vi "reconstruct 3D oblique image without config-2 (SubVI).vi"(0 "correction":T2={"vibration removal"=FALSE, "x correct fast/slow"=TRUE, "y correct fast/slow"=TRUE, "z correct fast/slow"=TRUE}, 1 "auto z adjust":T1={"margin"=100.0, "auto z adj"=FALSE, "average"=10, "use given ofst"=FALSE, "given ofst"=10}, 5 "image in":u16[][][](array[numeric])=array4x300x2304[2764800 elements], 7 "config in":T3={"xy cut pos correct"=[[0.0, 0.0, 0.0, 0.0], [0.0, 0.0, 0.0, 0.0], [0.0, 0.0, 0.0, 0.0], [0.0, 0.0, 0.0, 0.0], [0.0, 0.0, 0.0, 0.0], [0.0, 0.0, 0.0, 0.0], [0.0, 0.0, 0.0, 0.0], [0.0, 0.0, 0.0, 0.0], [0.0, 0.0, 0.0, 0.0], [0.0, 0.0, 0.0, 0.0], [0.0, 0.0, 0.0, 0.0], [0.0, 0.0, 0.0, 0.0], [0.0, 0.0, 0.0, 0.0], [0.0, 0.0, 0.0, 0.0], [0.0, 0.0, 0.0, 0.0], [0.0, 0.0, 0.0, 0.0], [0.0, 0.0, 0.0, 0.0], [0.0, 0.0, 0.0, 0.0], [0.0, 0.0, 0.0, 0.0], [0.0, 0.0, 0.0, 0.0], [0.0, 0.0, 0.0, 0.0], [0.0, 0.0, 0.0, 0.0], [0.0, 0.0, 0.0, 0.0], [0.0, 0.0, 0.0, 0.0]], "3D reconst config"={"xyz pos"=[46, 31, 52], "color 4"={"color array"=[0, 8388736, 16711680, 16776960, 16776960, 16711680, 16448250, 16448250], "num of colors"=4, "max"=7000.900000000023, "min"=100.0}, "autogain"=TRUE, "zoom"=1.0, "slice(T)/stack(F)"=FALSE, "xy cut mag"=0.9999999999999872, "xy cut ofst"=10.0, "z/xy comp"=0.9999999999999996, "y shift comp"=2.0, "max plot"=TRUE, "oblique angle [deg]"=45.0, "voxel size z [um]"=0.2909342537087903, "voxel size xy[um]"=0.20475, "reverse v"=FALSE, "reverse h"=TRUE, "3D reconstruction"=TRUE, "reverse z"=FALSE}, "xy cut pos"=[[0.0, 1.037506591193278, 0.966249270369417, 0.9158940969875857], [92.08631074928655, 92.74282819847565, 92.97750230838835, 92.67727146331777], [184.28758330950427, 185.01250778668418, 185.4134489785189, 184.69137479417213], [276.0489606758347, 276.53636075026884, 276.69217675847005, 276.4860055768869], [368.07921566607354, 368.89819980674065, 368.8136411193633, 368.38419699919905], [461.798744208641, 461.9849633403935, 462.2490904762467, 462.24814037863575], [554.7781467122519, 555.268397079519, 555.2332434679125, 554.7296917340917], [647.2882009960379, 647.5846314506646, 647.6995932615935, 647.5152743250628], [740.8889673372312, 741.2737568696792, 741.2034496464664, 740.8557139208467], [833.9643296995517, 834.1876026381326, 834.4726319214276, 834.3510194272217], [926.4886354475025, 926.7024074099736, 926.5560923778821, 926.5332900352184], [1019.2086613033152, 1019.556397028935, 1019.5734987859327, 1019.5449958576031], [1112.8274794991178, 1113.0498023400878, 1112.7296194451865, 1112.9329403339368], [1205.8866902020513, 1205.9931011344815, 1205.9531970348203, 1205.9037919590492], [1298.9126474886007, 1298.899346122047, 1299.058012423081, 1299.116918474962], [1392.299641867323, 1392.3689989929248, 1391.9509560440924, 1392.082069514408], [1485.6457820487744, 1485.6942370269344, 1485.3132478849304, 1485.3569523750357], [1578.3297041953701, 1578.9007128595708, 1578.61948396672, 1578.8503576861888], [1671.6273893986595, 1671.6549422293779, 1671.4050665576897, 1671.3604119699735], [1764.8661685500688, 1764.862368159625, 1764.8129630838534, 1765.1844512497485], [1857.8854751533427, 1857.8854751533427, 1857.6869047526473, 1857.7192080714206], [1951.1917112351302, 1951.1964617231852, 1951.2800703129517, 1951.4168843689333], [2043.5326481441634, 2043.787274303907, 2043.6352586861497, 2043.5982048793212], [2136.2422229262547, 2136.4265418627856, 2136.2099196074814, 2136.124410822493]], "AOD scan speed ratio"=5.0, "Nx"=93.5, "stack method"=enum."0pad to x and rot", "y shift"=3}, 9 "cropcalib":bool, 11 "cropcalib data":dbl[][][](array[numeric])=[[[330.8512624722854, 1176.151016996622, 0.0, 0.009428316830650669], [328.5787621076082, 1180.3546677235079, 0.0, 0.009179659527843352], [329.1155115826025, 1185.5118549945614, 0.0, 0.008879926465064643], [328.4474666338575, 1190.066406913501, 0.0, 0.00862012495571322]], [[327.58384877552515, 1179.3399452115818, 0.0, 0.009239326761173557], [330.64586772559215, 1183.570509586454, 0.0, 0.008992065492687374], [329.1182426075196, 1188.7090456628334, 0.0, 0.008697068994156926], [331.0833292234464, 1193.2988555935556, 0.0, 0.008438543533451089]], [[328.7041098476068, 1182.569513173517, 0.0, 0.009050212846350443], [330.5655883182281, 1186.770481635967, 0.0, 0.008807670479919528], [328.3880581820918, 1191.9068661319957, 0.0, 0.00851645191863399], [330.8192081039448, 1196.484526211637, 0.0, 0.008261875826756079]], [[329.0291138405168, 1185.8638941976924, 0.0, 0.00885968095793796], [330.2239592659729, 1190.0021055331606, 0.0, 0.008623760711384792], [329.88360431477196, 1195.207928124911, 0.0, 0.00833239920230058], [329.0055546600167, 1200.7794531816844, 0.0, 0.008027295813293513]], [[330.24527413712724, 1189.0833512123208, 0.0, 0.008675809944263788], [328.9577860583197, 1193.1902259931223, 0.0, 0.0084446078534114], [328.4487732377894, 1198.4548030016394, 0.0, 0.008153748883619465], [330.0763524036554, 1204.0443558848656, 0.0, 0.00785175048715124]], [[327.9606329363599, 1192.2041314919686, 0.0, 0.008499777889598343], [330.446114732459, 1196.4188076408827, 0.0, 0.008265497412007088], [331.55926553798633, 1201.6905041902264, 0.0, 0.007978069360316281], [330.71140004975507, 1207.1845836973916, 0.0, 0.0076851779540676735]], [[329.5691345378466, 1195.4239688330229, 0.0, 0.008320438746162742], [330.7306447795087, 1200.618390032539, 0.0, 0.008036017910836857], [329.65318996509365, 1204.906703846507, 0.0, 0.007805785611196943], [330.4225359020906, 1210.364940978633, 0.0, 0.0075187501899264125]], [[328.35008836956763, 1198.6407415088522, 0.0, 0.008143589762204376], [328.90402303435104, 1203.8024115267247, 0.0, 0.007864676757548733], [328.8872850578613, 1208.09777539, 0.0, 0.007637156351356103], [328.3105695920642, 1213.5593257233536, 0.0, 0.007353896502053807]], [[328.6451967358637, 1127.9703327325547, 0.0, 0.012550072767244045], [328.19424909379455, 1133.085548853325, 0.0, 0.012195479564778025], [328.3679132256721, 1137.3419122345406, 0.0, 0.011904528149263727], [329.8664011804312, 1142.824068114119, 0.0, 0.011535328382056603]], [[329.0137931176627, 1131.1684730544375, 0.0, 0.012327745071188015], [329.43921945403974, 1136.330837065185, 0.0, 0.011973302642268695], [330.07216132208566, 1140.623130285924, 0.0, 0.01168279908476291], [328.1737251840431, 1145.9867948563115, 0.0, 0.0113251919030582]], [[330.1899355869486, 1134.39359452557, 0.0, 0.012105667313626528], [328.70790882861525, 1139.5021004338992, 0.0, 0.011758300895061025], [328.0782246591683, 1143.8377820926603, 0.0, 0.01146774697568997], [329.54950432096183, 1149.2241857413321, 0.0, 0.011112275930991233]], [[331.42214147724894, 1137.5528595644162, 0.0, 0.011890206002647927], [330.97763687982894, 1142.7297019826956, 0.0, 0.01154163045813605], [330.54961412343954, 1147.0781334797975, 0.0, 0.011253169866028413], [327.0844397044803, 1152.4396225757132, 0.0, 0.010902999394719153]], [[330.929575643222, 1140.7785447879169, 0.0, 0.011672352543176941], [328.8439266492678, 1145.8708900077258, 0.0, 0.011332855690938066], [331.16506613573154, 1151.328789104024, 0.0, 0.010975049855985547], [332.3144635692056, 1155.6809834714056, 0.0, 0.010694261336075706]], [[328.87791169340977, 1143.9447348598565, 0.0, 0.011460629308520941], [328.60841680034633, 1149.0313226737098, 0.0, 0.011124898082049313], [328.28437086297305, 1154.4927373292637, 0.0, 0.010770522200949609], [327.16287039111825, 1158.8764418635192, 0.0, 0.010490677347170251]], [[329.35729265333816, 1147.090501489575, 0.0, 0.011252355087675737], [328.14957842477327, 1152.2634326180323, 0.0, 0.010914409859878342], [328.4917513371784, 1157.727572410442, 0.0, 0.01056362038447542], [330.95966686347083, 1162.1495563864858, 0.0, 0.01028441907635147]], [[329.1515568019215, 1151.3685299195897, 0.0, 0.010972467680426496], [332.2082161856812, 1155.482901454856, 0.0, 0.010706953165264467], [329.86557476312265, 1160.9761057095386, 0.0, 0.010358099929698581], [326.6180198128402, 1165.2756124065388, 0.0, 0.010089585308586238]], [[328.2018949478854, 1154.6071079334506, 0.0, 0.010763168859236505], [326.6757431393615, 1158.6721466023419, 0.0, 0.010503627582312526], [329.0019237207534, 1164.24453850444, 0.0, 0.010153614215199027], [330.29906981784274, 1168.5264642776929, 0.0, 0.009889219147039267]], [[330.7756952264671, 1157.893428641218, 0.0, 0.010553072495697563], [331.7656713031102, 1161.921777606122, 0.0, 0.010298698065293217], [328.3819521167621, 1167.4401073598385, 0.0, 0.00995592141258132], [329.42308717648444, 1171.686971815366, 0.0, 0.009696625521530881]], [[330.0486596989607, 1161.1143527630184, 0.0, 0.0103494039902354], [329.1844277898541, 1165.0713046949666, 0.0, 0.01010225437575639], [328.8711921864445, 1170.6878812751677, 0.0, 0.009757272221675928], [330.1502018730359, 1175.9537054449938, 0.0, 0.009440083845015646]], [[330.0279911009871, 1164.3021214095252, 0.0, 0.01015003229395419], [328.95127385724874, 1168.2935980154227, 0.0, 0.009903495516852285], [328.85226629139345, 1173.9565370919474, 0.0, 0.009559669235622265], [328.60848310183206, 1179.144742459143, 0.0, 0.009250831019732907]], [[329.797813873803, 1167.4416972495085, 0.0, 0.00995582360599151], [330.2854633911041, 1171.5422434795005, 0.0, 0.009705397308885887], [328.7652670570403, 1177.1705548368723, 0.0, 0.009367651211476397], [329.8191554231605, 1182.350456061726, 0.0, 0.009062967328391715]], [[328.76403530096667, 1170.631972332091, 0.0, 0.009760672437718717], [328.55523679710865, 1175.8083846400932, 0.0, 0.00944875576806857], [331.14545931703805, 1180.3934166639754, 0.0, 0.00917738553352469], [330.6972097456994, 1185.5925133499545, 0.0, 0.008875285435237572]], [[330.6527669048852, 1173.9082717155898, 0.0, 0.00956257006524093], [329.370737307894, 1179.0415869795693, 0.0, 0.009256913871127877], [330.81783725373816, 1183.6004158389724, 0.0, 0.008990331666880891], [328.0387873941186, 1188.7560952119093, 0.0, 0.008694395054772111]], [[327.27231388978987, 1177.0924704019544, 0.0, 0.0093722893955023], [329.7294177817484, 1182.2906875157555, 0.0, 0.009066449162680675], [328.797293940435, 1186.8506176880321, 0.0, 0.008803081896203244], [328.1656445749852, 1191.9915781247635, 0.0, 0.008511698293876373]]], 12 "array":i32[](array[numeric]), 13 "create 2D img":bool=TRUE) -> (2 "voxel number":i32[](array[numeric])=[65, 299, 203], 3 "image size":dbl[](array[numeric])=[65.0, 299.0, 203.0], 4 "z ofst":dbl, 6 "combined img2":u16[][](array[numeric]), 8 "xyz2":u16[][][](array[numeric]), 10 "voxel size [um]":dbl[](array[numeric])=[0.20475, 0.20475, 0.20475], 14 "combined img":u16[][](array[numeric]), 15 "xyz":u16[][][](array[numeric]))   [LabVIEW 2024]
uses:
  Global variables/global for picoscope.vi
  <vilib>/gmath/NI_Gmath.lvlib
panel:
  out "x-y 9":dbl=0.20982419996289536
  out "x-y 8":dbl=0.09279239998431876
  out "x-y 7":dbl=0.20982419996289536
  out "x-y 5":dbl=0.20982419996289536
  out "element":i32=24
  in  "spacing":i32=10
  out "x-y 3":dbl=0.09279239998431876
  out "Intensity Graph 3":u16[][](graph)
  out "Intensity Graph 2":u16[][](graph)
  out "Intensity Graph":u16[][](graph)
  out "x-y 2":dbl=0.20982419996289536
  out "x-y":dbl=0.38623420003568754
  out "frame's init pos in x":dbl[][](array[numeric])=[[0.0, 3.6829999999999927, 4.111999999999966, 4.5049999999999955], [208.139, 211.894, 212.505, 212.31799999999998], [423.026, 426.562, 427.187, 427.31300000000005], [643.657, 646.902, 647.605, 647.8430000000001], [872.2024, 875.6199, 876.0371, 876.0722000000001], [1107.138, 1110.396, 1110.987, 1111.045], [1345.127, 1348.448, 1348.937, 1349.342], [1578.719, 1581.7530000000002, 1582.527, 1583.004], [1797.017, 1800.116, 1800.629, 1800.951], [1984.0770000000002, 1986.647, 1987.3670000000002, 1988.147]]
  out "zy":u16[][](array[numeric])
  out "zx":u16[][](array[numeric])
  out "yx":u16[][](array[numeric])
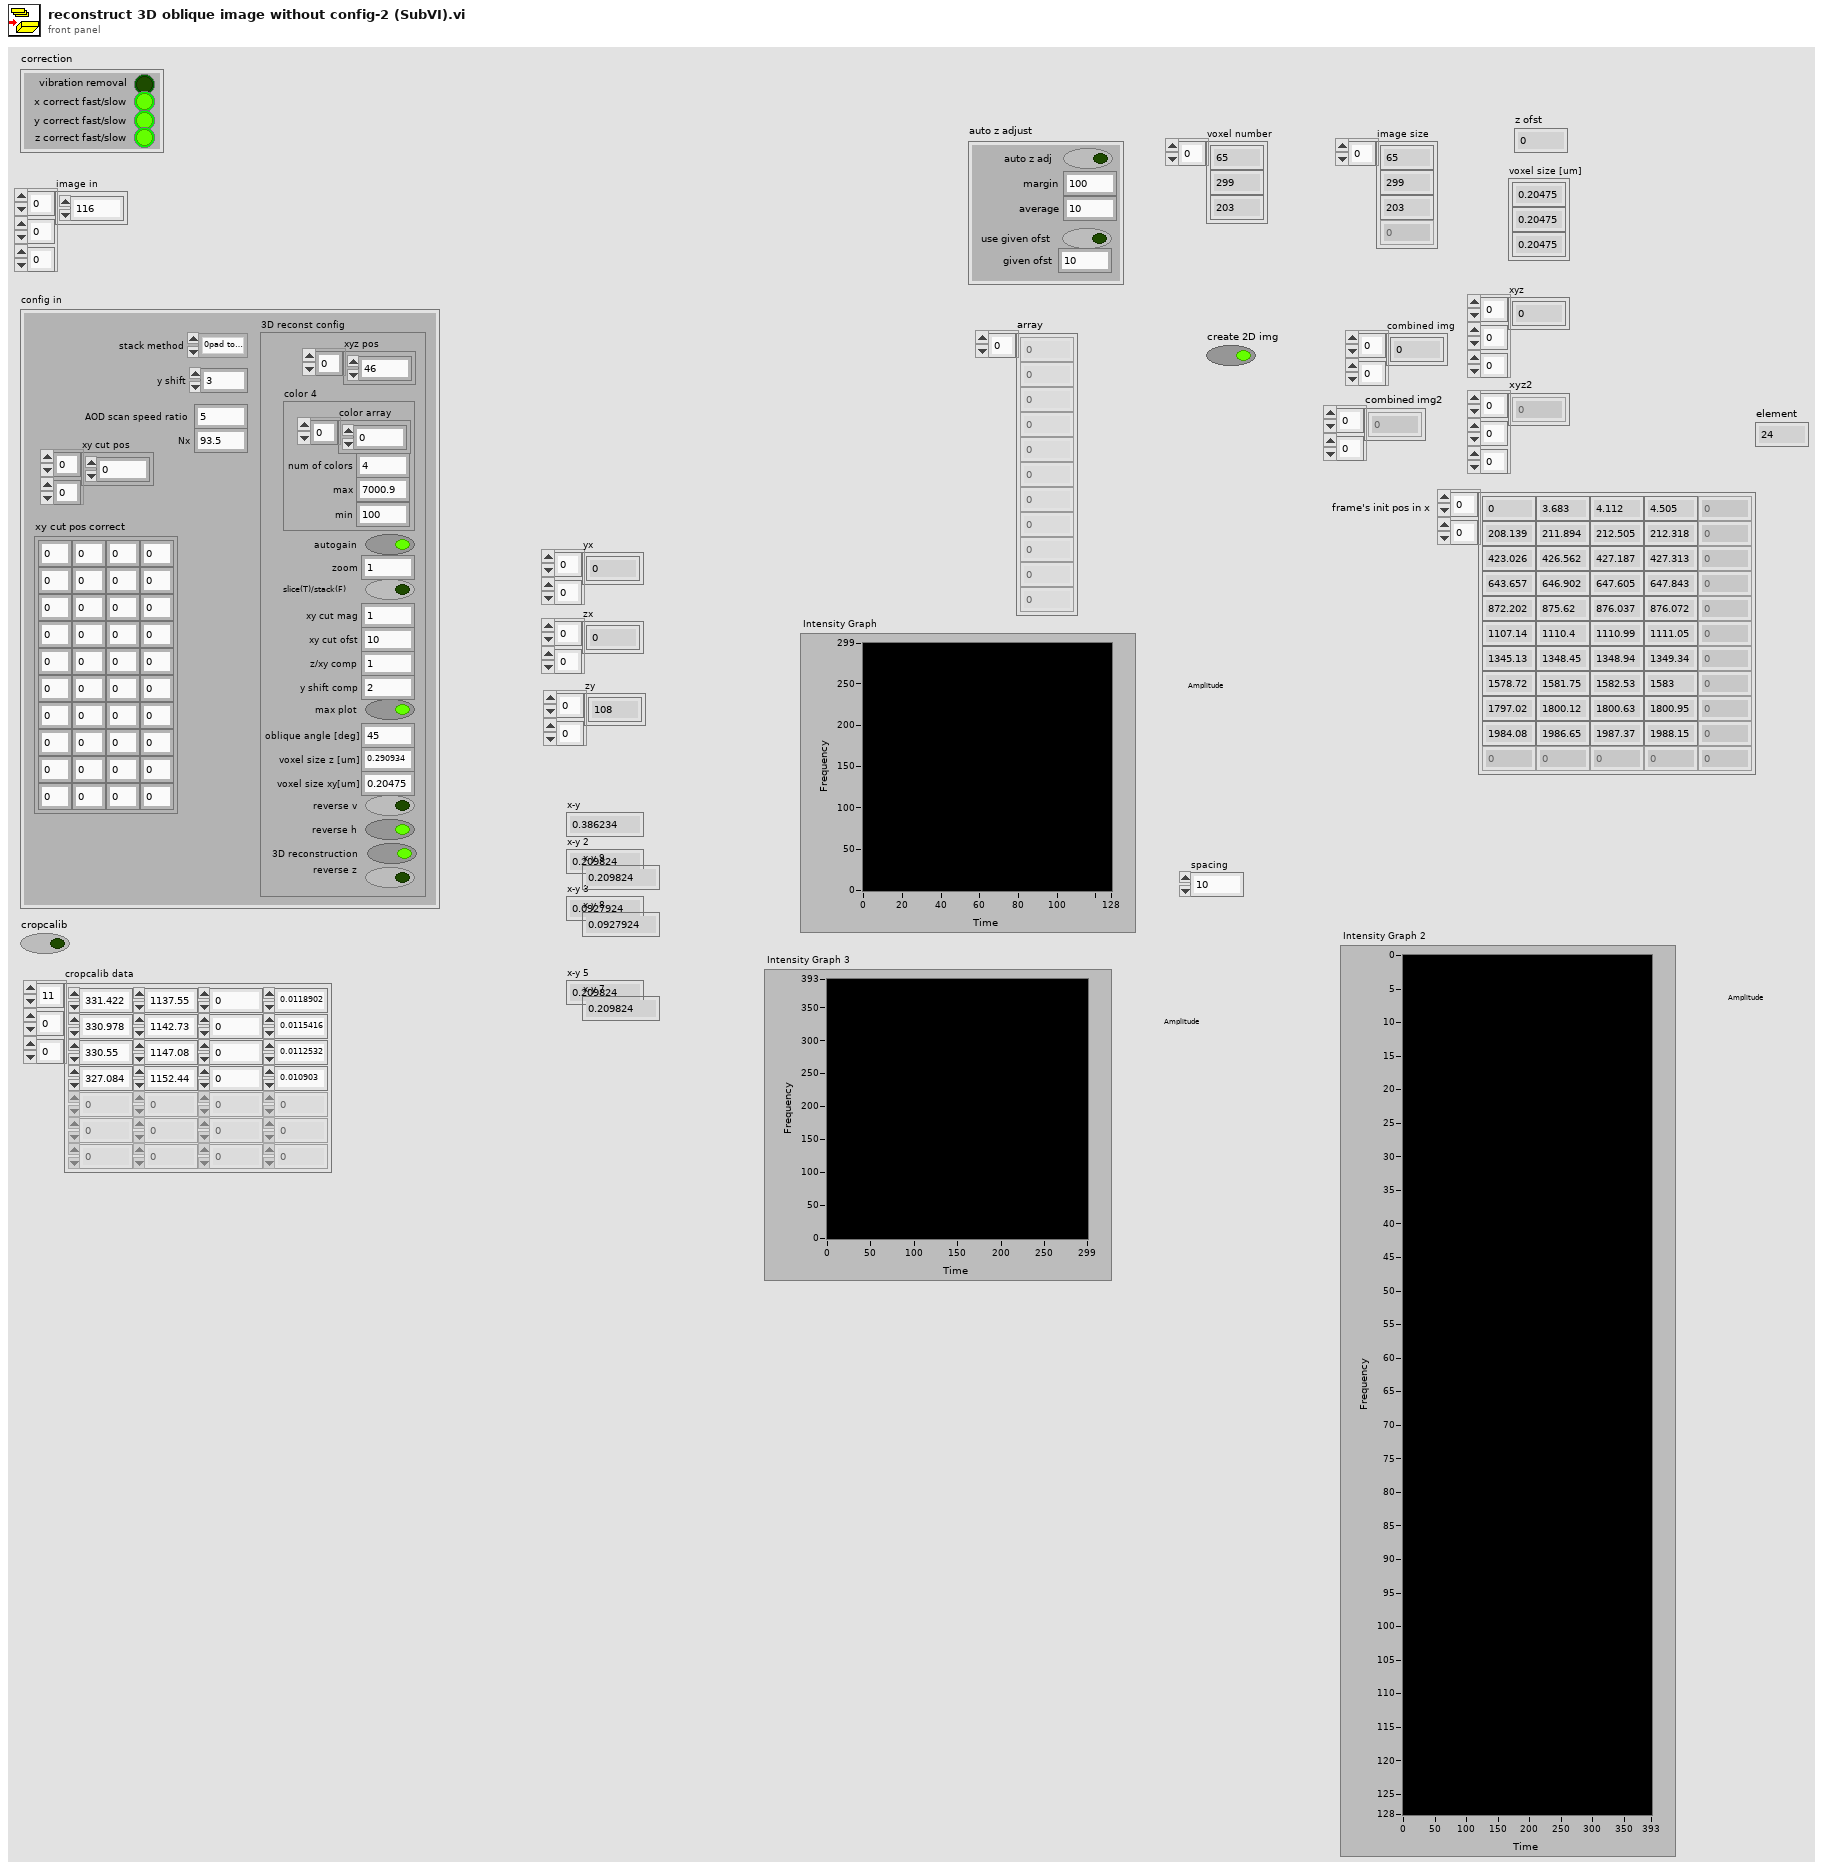
[diagram p1: front panel]
types:
  T1 = cluster{"margin":dbl, "auto z adj":bool, "average":i32, "use given ofst":bool, "given ofst":i32}
  T2 = cluster{"vibration removal":bool, "x correct fast/slow":bool, "y correct fast/slow":bool, "z correct fast/slow":bool}
  T3 = cluster{"xy cut pos correct":dbl[][], "3D reconst config":cluster{"xyz pos":u16[], "color 4":cluster{"color array":u32[], "num of colors":i32, "max":dbl, "min":dbl}, "autogain":bool, "zoom":dbl, "slice(T)/stack(F)":bool, "xy cut mag":dbl, "xy cut ofst":dbl, "z/xy comp":dbl, "y shift comp":dbl, "max plot":bool, "oblique angle [deg]":dbl, "voxel size z [um]":dbl, "voxel size xy[um]":dbl, "reverse v":bool, "reverse h":bool, "3D reconstruction":bool, "reverse z":bool}, "xy cut pos":dbl[][], "AOD scan speed ratio":dbl, "Nx":dbl, "stack method":enum16{"0pad to z", "0pad to x", "0pad to x and rot", "none"}, "y shift":i32}
  T4 = cluster{"xyz pos":u16[], "color 4":cluster{"color array":u32[], "num of colors":i32, "max":dbl, "min":dbl}, "autogain":bool, "zoom":dbl, "slice(T)/stack(F)":bool, "xy cut mag":dbl, "xy cut ofst":dbl, "z/xy comp":dbl, "y shift comp":dbl, "max plot":bool, "oblique angle [deg]":dbl, "voxel size z [um]":dbl, "voxel size xy[um]":dbl, "reverse v":bool, "reverse h":bool, "3D reconstruction":bool, "reverse z":bool}
  T5 = enum16{"0pad to z", "0pad to x", "0pad to x and rot", "none"}
  T6 = enum16{"no change", "zyx->zxy", "zyx->xyz", "zyx->yzx", "zyx->yxz", "zyx->xzy"}
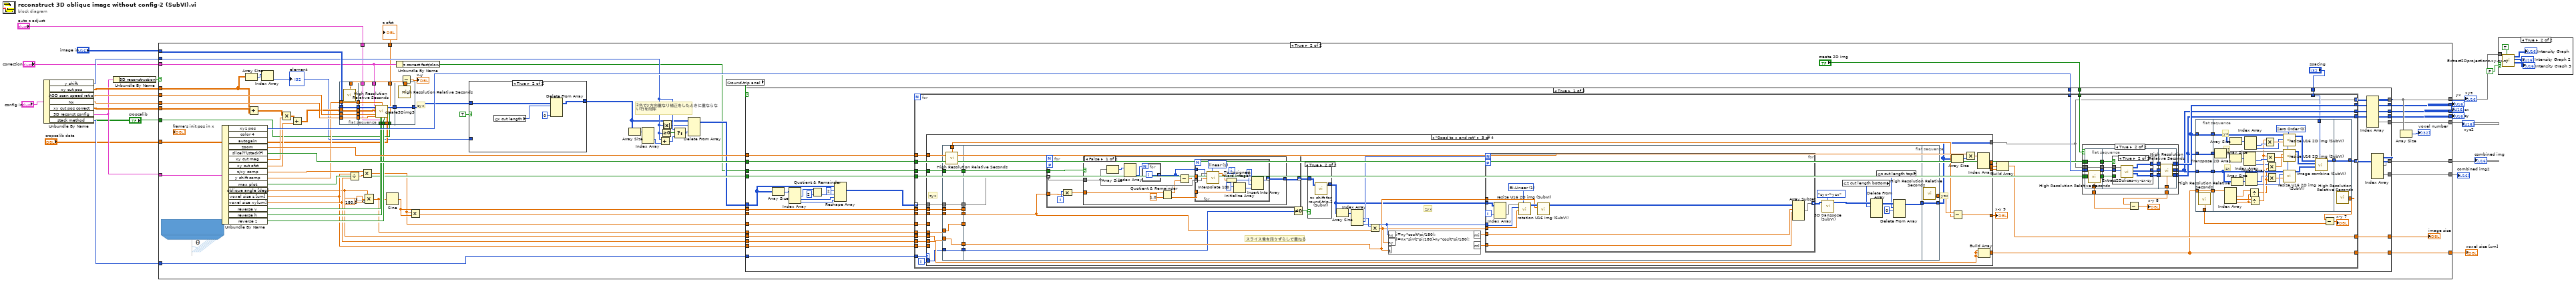
[diagram p0: block diagram]
diagram:
  n1 = Unbundle By Name("config in") -> ("y shift"=w15:i32, "xy cut pos"=w14:dbl[][], "AOD scan speed ratio"=w13:dbl, "Nx"=w12:dbl, "xy cut pos correct"=w11:dbl[][], "3D reconst config"=w10:T4, "stack method"=w9:T5)
  n2 = Unbundle By Name(w10) -> ("3D reconstruction"=w24:bool)
  n3 = case shown="True" w24 {
    tunnel: w12 -> [_ w97]
    tunnel: w13 -> [_ w96]
    tunnel: "image in" -> [_ w90]
    tunnel: w14 -> [_ w45]
    tunnel: w10 -> [_ w89]
    tunnel: [_ w52] -> w20
    tunnel: [_ w37] -> w21
    tunnel: [_ w53] -> w22
    tunnel: [_ w58] -> w19
    tunnel: [_ w51] -> w17
    tunnel: w11 -> [_ w56]
    tunnel: w15 -> [_ w55]
    tunnel: w9 -> [_ w54]
    tunnel: [_ w50] -> w8
    tunnel: "cropcalib" -> [_ w49]
    tunnel: "cropcalib data" -> [_ w48]
    tunnel: "correction" -> [_ w42]
    tunnel: [0.0 ("z ofst") w39] -> w4
    tunnel: "auto z adjust" -> [_ w38]
    tunnel: [_ w35] -> w2
    tunnel: [_ w33] -> w1
    frame False {
    }
    frame True {
      # "2色でy方向重なり補正をしたときに重ならない行を削除"
      # "zyx"
      n4 = Unbundle By Name(w89) -> ("xyz pos"=w88:u16[], "zoom"=w87:dbl, "slice(T)/stack(F)"=w86:bool, "xy cut mag"=w85:dbl, "xy cut ofst"=w77:dbl, "z/xy comp"=w84:dbl, "y shift comp"=w79:dbl, "max plot"=w80:bool, "oblique angle [deg]"=w61:dbl, "voxel size z [um]"=w65:dbl, "voxel size xy[um]"=w66:dbl, "reverse v"=w82:bool, "reverse h"=w83:bool, "reverse z"=w81:bool)  [unwired: 2 out]
      n5 = Array Size(array=w45) -> (size(s)=w44:i32[])
      n6 = Add(x=w56, y=w45) -> (x+y=w94:dbl[][])
      n7 = Index Array(array=w44) -> (element=w43:i32)  [unwired: 1 in]
      "element" <- w43
      n8 = Multiply(x=w94, y=w85) -> (x*y=w78:dbl[][])
      n9 = Add(x=w78, y=w77) -> (x+y=w95:dbl[][])
      n10 = flat-sequence {
        tunnel: w79 -> [w897]
        tunnel: w90 -> [w898]
        tunnel: w95 -> [w899]
        tunnel: w96 -> [w900]
        tunnel: w97 -> [w901]
        tunnel: [w901] -> w76
        tunnel: [w900] -> w75
        tunnel: [w899] -> w74
        tunnel: [w898] -> w73
        tunnel: [w897] -> w72
        tunnel: [w896] -> w69
        tunnel: w83 -> [w911]
        tunnel: w82 -> [w910]
        tunnel: w81 -> [w909]
        tunnel: w76 -> [w915]
        tunnel: w75 -> [w914]
        tunnel: w74 -> [w913]
        tunnel: w73 -> [w912]
        tunnel: w72 -> [w908]
        tunnel: [w905] -> w71
        tunnel: w49 -> [w907]
        tunnel: w48 -> [w906]
        tunnel: w42 -> [w904]
        tunnel: [w903] -> w39
        tunnel: w38 -> [w902]
        tunnel: [w917] -> w47
        tunnel: w71 -> [w917]
        tunnel: [w916] -> w70
        frame #0 {
          n11 = call <vilib>:"High Resolution Relative Seconds.vi"() -> ("relative seconds"=w896:dbl)
        }
        frame #1 {
          n12 = call "create3Dimg3.vi"("input"=w912, "reverse y"=w910, "v comp"=w908, "x init pos"=w913, "correction"=w904, "AOD scan speed ratio"=w914, "cropcalib"=w907, "Nx"=w915, "reverse x"=w911, "auto z adjust"=w902, "reverse z"=w909, "cropcalib data"=w906) -> ("zyx"=w905:u16[][][], "z ofst"=w903:dbl)  [unwired: 2 in]
        }
        frame #2 {
          n13 = call <vilib>:"High Resolution Relative Seconds.vi"() -> ("relative seconds"=w916:dbl)
        }
      }
      n14 = Divide(x=w65, y=w66) -> (x/y=w91:dbl)
      n15 = Multiply(x=w84, y=w91) -> (x*y=w63:dbl)
      n16 = Compound Arithmetic op=MULTIPLY(w61, 3.141592653589793, invert 180.0) -> (w67:dbl)
      n17 = Sine(x=w67) -> (sin(x)=w64:dbl)
      n18 = Unbundle By Name(w42) -> ("z correct fast/slow"=w41:bool)
      n19 = Subtract(x=w70, y=w69) -> (x-y=→"x-y":dbl)
      n20 = Multiply(x=w63, y=w64) -> (x*y=w62:dbl)
      n21 = case shown="True" TRUE {
        tunnel: w47 -> [w100 w119]
        tunnel: [w99 w117] -> w46
        tunnel: w43 -> [w98 _]
        frame False {
          n22 = for {
            tunnel: w100 -> [w106] mode=indexing
            tunnel: [w107] -> w99 mode=indexing
            tunnel: w98 -> [w101]
            i -> [w102]
            # "はみ出た隣接スライス像を除去"
            n23 = Array Size(array=w106) -> (size(s)=w109:i32[])
            n24 = Index Array(array=w109) -> (element=w110:i32)  [unwired: 1 in]
            n25 = Quotient & Remainder(x=w102, y=w101) -> (x-y*floor(x/y)=w105:i32)  [unwired: 1 out]
            n26 = Index Array(array="array", index=w105) -> (element=w104:i32)
            n27 = Initialize Array(u16 100, w110) -> (w111:u16[])
            n28 = for {
              N: w104 -> [_]
              tunnel: w111 -> [w115]
              shift-right: [w114] -> w107
              shift-left: w106 -> [w112]
              i -> [w113]
              n29 = Replace Array Subset(array=w112, new element=w115, index (col)=w113) -> (w114:u16[][])  [unwired: 1 in]
            }
          }
        }
        frame True {
          n30 = global read "global for picoscope.vi" "x cut length"() -> (w116:u32)
          n31 = Delete From Array(array=w119, length=w116, index (dim 2)=0 ("index (col)")) -> (array with subset deleted=w117:u16[][][])  [unwired: 2 in, 1 out]
        }
      }
      n32 = Array Size(array=w46) -> (size(s)=w32:i32[])
      n33 = Index Array(array=w32) -> (element #2=w27:i32)  [unwired: 3 in, 2 out]
      n34 = Add(x=w55, y=w27) -> (x+y=w28:i32)
      n35 = Greater Or Equal To 0?(x=w55) -> (x >= 0?=w29:bool)
      n36 = Absolute Value(x=w55) -> (abs(x)=w31:i32)
      n37 = Select(t=w55, s=w29, f=w28) -> (s? t:f=w30:i32)
      n38 = Delete From Array(array=w46, length=w31, index (dim 1)=w30) -> (array with subset deleted=w59:u16[][][])  [unwired: 2 in, 1 out]
      n39 = global read "global for picoscope.vi" "round-trip anal"() -> (w36:bool)
      n40 = case shown="True" w36 {
        tunnel: w88 -> [w154 w568]
        tunnel: w87 -> [w153 w567]
        tunnel: w86 -> [w152 w566]
        tunnel: w80 -> [w151 w565]
        tunnel: w67 -> [w150 w563]
        tunnel: w66 -> [w149 w562]
        tunnel: w65 -> [w148 w561]
        tunnel: w64 -> [w147 w560]
        tunnel: w63 -> [w146 w559]
        tunnel: w62 -> [w145 w558]
        tunnel: w61 -> [w144 w557]
        tunnel: [w143 w553] -> w60
        tunnel: w59 -> [w131 w549]
        tunnel: [w126 w548] -> w58
        tunnel: w54 -> [w141 w547]
        tunnel: [w140 w546] -> w53
        tunnel: [w139 w545] -> w52
        tunnel: [w138 w544] -> w51
        tunnel: [w122 w543] -> w50
        tunnel: w41 -> [w137 w542]
        tunnel: "create 2D img" -> [w136 w541]
        tunnel: [w135 w537] -> w37
        tunnel: [w125 _] -> w35
        tunnel: "spacing" -> [w124 w536]
        tunnel: [w121 _] -> w33
        frame True {
          n41 = Array Size(array=w131) -> (size(s)=w133:i32[])
          n42 = Index Array(array=w133) -> (element #1=w132:i32, element #2=w128:i32, element #3=w127:i32)  [unwired: 3 in]
          n43 = Quotient & Remainder(x=w132, y=2) -> (floor(x/y)=w129:i32)  [unwired: 1 out]
          n44 = Reshape Array(w131, 2 ("dimension size"), w129, w128, w127) -> (w120:u16[][][][])
          n45 = for {
            tunnel: w154 -> [w188]
            tunnel: w153 -> [w187]
            tunnel: w152 -> [w186]
            tunnel: w151 -> [w185]
            tunnel: w150 -> [w183]
            tunnel: w149 -> [w182]
            tunnel: w148 -> [w181]
            tunnel: w147 -> [w180]
            tunnel: w146 -> [w179]
            tunnel: w145 -> [w178]
            tunnel: w144 -> [w177]
            tunnel: [w173] -> w143
            tunnel: [w155] -> w142 mode=indexing
            tunnel: w141 -> [w169]
            tunnel: [w168] -> w140
            tunnel: [w167] -> w139
            tunnel: [w166] -> w138
            tunnel: [w165] -> w123 mode=indexing
            tunnel: w137 -> [w164]
            tunnel: w136 -> [w163]
            tunnel: [w159] -> w135
            tunnel: w120 -> [w158] mode=indexing
            tunnel: w124 -> [w157]
            i -> [w156]
            n46 = case shown="\"0pad to x and rot\"" w169 {
              tunnel: w158 -> [w272 w358 w439 w535]
              tunnel: w179 -> [_ w342 _ _]
              tunnel: [w278 w347 w424 w534] -> w176
              tunnel: [w279 w354 w436 w532] -> w174
              tunnel: [w287 w353 w435 w533] -> w175
              tunnel: w187 -> [w289 w352 w434 _]
              tunnel: [w285 w334 w425 w535] -> w155
              tunnel: [w284 w349 w431 _] -> w184
              tunnel: w183 -> [w282 w341 w429 _]
              tunnel: w182 -> [w275 w344 w420 w531]
              tunnel: w181 -> [w276 w345 _ w528]
              tunnel: w180 -> [_ _ w427 _]
              tunnel: w178 -> [_ _ w426 _]
              tunnel: w177 -> [_ _ w422 _]
              tunnel: [w273 w343 w421 w530] -> w166
              tunnel: w164 -> [_ w338 w418 _]
              tunnel: w156 -> [_ w333 w416 _]
              frame "0pad to z", Default {
                # "voxel size\npx sint\npy\npx sint"
                # "ZYX=xyz xとzが入れ替わっている"
                n47 = flat-sequence {
                  tunnel: w272 -> [w300]
                  tunnel: [w300] -> w295
                  tunnel: [w299] -> w290
                  tunnel: [w298] -> w283
                  tunnel: w282 -> [w298]
                  tunnel: [w297] -> w281
                  tunnel: w275 -> [w297]
                  tunnel: [w296] -> w280
                  tunnel: w276 -> [w296]
                  tunnel: w295 -> [w303]
                  tunnel: [w301] -> w294
                  tunnel: w283 -> [w310]
                  tunnel: w281 -> [w308]
                  tunnel: w280 -> [w309]
                  tunnel: [w302] -> w277
                  tunnel: [w332] -> w285
                  tunnel: w294 -> [w332]
                  tunnel: [w331] -> w291
                  frame #0 {
                    n48 = call <vilib>:"High Resolution Relative Seconds.vi"() -> ("relative seconds"=w299:dbl)
                  }
                  frame #1 {
                    # "xyz=ZYX\nZは真の奥行方向"
                    # "zyx"
                    n49 = Sine(x=w310) -> (sin(x)=w302:dbl)
                    n50 = Array Size(array=w303) -> (size(s)=w311:i32[])
                    n51 = Index Array(array=w311) -> (element #1=w305:i32, element #2=w304:i32, element #3=w306:i32)  [unwired: 3 in]
                    n52 = Compound Arithmetic op=MULTIPLY(w305, w309, invert w302, invert w308) -> (w307:dbl)
                    n53 = for {
                      N: w306 -> [w315]
                      tunnel: w303 -> [w322]
                      tunnel: [w316] -> w301 mode=indexing
                      workers-P: _ -> [_]
                      tunnel: w304 -> [w317]
                      tunnel: w307 -> [w318]
                      i -> [w313]
                      w319 = u32 0 items=["Zero Order", "Bi-Linear", "Quadratic", "Cubic Spline"] ("Interpolation Type")
                      # "yz"
                      # "zピクセルサイズをxsinθにする"
                      # "yzスライス像を段々ずらしで重ねる"
                      # "zy"
                      n54 = Decrement(x=w315) -> (x-1=w314:i32)
                      n55 = Subtract(x=w314, y=w313) -> (x-y=w312:i32)
                      n56 = Index Array(array=w322, index (dim 2)=w312) -> (element=w321:u16[][])  [unwired: 2 in]
                      n57 = call "resize U16 2D img (SubVI).vi"("Interpolation Type"=w319, "Y Resolution"=w318, "X Resolution"=w317, "Array"=w321) -> ("Image Pixels (U16)"=w320:u16[][])  [unwired: 7 in]
                      n58 = for {
                        N: w317 -> [_]
                        tunnel: w320 -> [w330]
                        tunnel: [w326] -> w316 mode=indexing
                        tunnel: w312 -> [w325]
                        i -> [w323]
                        # "z"
                        n59 = Index Array(array=w330, index (col)=w323) -> (element=w324:u16[])  [unwired: 1 in]
                        n60 = Initialize Array(u16 0 ("element"), w325) -> (w327:u16[])
                        n61 = Insert Into Array(array=w324, index=0, new element=w327) -> (w326:u16[])
                      }
                    }
                  }
                  frame #2 {
                    n62 = call <vilib>:"High Resolution Relative Seconds.vi"() -> ("relative seconds"=w331:dbl)
                  }
                }
                n63 = Subtract(x=w291, y=w290) -> (x-y=w284:dbl)
                n64 = Array Size(array=w285) -> (size(s)=w293:i32[])
                n65 = Multiply(x=w289, y=w293) -> (x*y=w292:dbl[])
                n66 = Multiply(x=w275, y=w277) -> (x*y=w274:dbl)
                n67 = Index Array(array=w292) -> (element #1=w288:dbl, element #2=w287:dbl, element #3=w286:dbl)  [unwired: 3 in]
                n68 = Multiply(x=w277, y=w286) -> (x*y=w279:dbl)
                n69 = Multiply(x=w288, y=w277) -> (x*y=w278:dbl)
                n70 = Build Array(w274, w275, w274) -> (w273:dbl[])
              }
              frame "0pad to x" {
                # "スライス像を段々ずらしで重ねる"
                # "zyx"
                # "zyx"
                n71 = Cosine(x=w341) -> (cos(x)=w339:dbl)
                n72 = Multiply(x=w345, y=w339) -> (x*y=w340:dbl)
                n73 = flat-sequence {
                  tunnel: w342 -> [w368]
                  tunnel: w358 -> [w369]
                  tunnel: [w369] -> w361
                  tunnel: [w368] -> w360
                  tunnel: [w367] -> w350
                  tunnel: [w366] -> w348
                  tunnel: w341 -> [w366]
                  tunnel: w338 -> [w365]
                  tunnel: [w365] -> w337
                  tunnel: w361 -> [w375]
                  tunnel: w360 -> [w373]
                  tunnel: [w374] -> w359
                  tunnel: w348 -> [w372]
                  tunnel: [w371] -> w346
                  tunnel: w337 -> [w370]
                  tunnel: [w415] -> w335
                  tunnel: w359 -> [w415]
                  tunnel: [w414] -> w351
                  frame #0 {
                    n74 = call <vilib>:"High Resolution Relative Seconds.vi"() -> ("relative seconds"=w367:dbl)
                  }
                  frame #1 {
                    n75 = Sine(x=w372) -> (sin(x)=w371:dbl)
                    n76 = for {
                      tunnel: w375 -> [w382] mode=indexing
                      tunnel: w373 -> [w380]
                      tunnel: [w379] -> w374 mode=indexing
                      tunnel: w371 -> [w378]
                      tunnel: w370 -> [w377]
                      workers-P: _ -> [_]
                      i -> [w381]
                      n77 = Compound Arithmetic op=MULTIPLY(w380, w381, w378) -> (w376:dbl)
                      n78 = case shown="False" w377 {
                        tunnel: w382 -> [w388 w407]
                        tunnel: w376 -> [w392 w406]
                        tunnel: [w389 w405] -> w379
                        frame False {
                          n79 = Array Size(array=w388) -> (size(s)=w387:i32[])
                          n80 = Index Array(array=w387) -> (element #2=w386:i32)  [unwired: 2 in, 1 out]
                          n81 = for {
                            N: w386 -> [_]
                            tunnel: [w393] -> w384 mode=indexing
                            i -> [w393]
                          }
                          n82 = Quotient & Remainder(x=w392, y=1.0) -> (x-y*floor(x/y)=w385:dbl, floor(x/y)=w390:dbl)
                          n83 = Subtract(x=w384, y=w385) -> (x-y=w383:dbl[])
                          n84 = for {
                            tunnel: w388 -> [w399] mode=indexing
                            tunnel: w390 -> [w402]
                            tunnel: [w400] -> w389 mode=indexing
                            tunnel: w384 -> [w398]
                            tunnel: w383 -> [w397]
                            w396 = 2 items=["nearest", "linear", "spline", "cubic Hermite", "Lagrange"] ("method")
                            n85 = call <vilib>:"Interpolate 1D.vi"("method"=w396, "xi"=w397, "X"=w398, "Y"=w399) -> ("yi"=w395:dbl[])  [unwired: 5 in, 2 out]
                            n86 = To Unsigned Word Integer(number=w395) -> (unsigned 16bit integer=w394:u16[])
                            n87 = Initialize Array(u16 0 ("element"), w402) -> (w401:u16[])
                            n88 = Insert Into Array(array=w394, index=0, new element=w401) -> (w400:u16[])
                          }
                        }
                        frame True {
                          n89 = for {
                            tunnel: w407 -> [w413] mode=indexing
                            tunnel: w406 -> [w410]
                            tunnel: [w408] -> w405 mode=indexing
                            n90 = Initialize Array(u16 0 ("element"), w410) -> (w409:u16[])
                            n91 = Insert Into Array(array=w413, index=0, new element=w409) -> (w408:u16[])
                          }
                        }
                      }
                    }
                  }
                  frame #2 {
                    n92 = call <vilib>:"High Resolution Relative Seconds.vi"() -> ("relative seconds"=w414:dbl)
                  }
                }
                n93 = Subtract(x=w351, y=w350) -> (x-y=w349:dbl)
                n94 = Not Equal To 0?(x=w333) -> (x != 0?=w336:bool)
                n95 = case shown="True" w336 {
                  tunnel: w335 -> [w362 w364]
                  tunnel: [w362 w363] -> w334
                  frame False {
                  }
                  frame True {
                    n96 = call "zx shift for round-trip-2 (SubVI).vi"("input"=w364) -> ("output"=w363:u16[][][])  [unwired: 10 in]
                  }
                }
                n97 = Array Size(array=w334) -> (size(s)=w357:i32[])
                n98 = Multiply(x=w352, y=w357) -> (x*y=w356:dbl[])
                n99 = Index Array(array=w356) -> (element #1=w355:dbl, element #2=w353:dbl, element #3=w354:dbl)  [unwired: 3 in]
                n100 = Compound Arithmetic op=MULTIPLY(w346, w342, w355) -> (w347:dbl)
                n101 = Build Array(w340, w344, w344) -> (w343:dbl[])
              }
              frame "0pad to x and rot" {
                # "yzx"
                # "zyx"
                n102 = flat-sequence {
                  tunnel: w426 -> [w449]
                  tunnel: w439 -> [w450]
                  tunnel: [w450] -> w442
                  tunnel: [w449] -> w441
                  tunnel: [w448] -> w432
                  tunnel: [w447] -> w430
                  tunnel: w429 -> [w447]
                  tunnel: [w446] -> w428
                  tunnel: w427 -> [w446]
                  tunnel: [w445] -> w423
                  tunnel: w422 -> [w445]
                  tunnel: [w444] -> w419
                  tunnel: w418 -> [w444]
                  tunnel: [w443] -> w417
                  tunnel: w416 -> [w443]
                  tunnel: w442 -> [w463]
                  tunnel: w441 -> [w462]
                  tunnel: [w453] -> w440
                  tunnel: w430 -> [_]
                  tunnel: w428 -> [_]
                  tunnel: w423 -> [w464]
                  tunnel: w419 -> [w461]
                  tunnel: w417 -> [w458]
                  tunnel: [w527] -> w425
                  tunnel: w440 -> [w527]
                  tunnel: [w526] -> w433
                  frame #0 {
                    n103 = call <vilib>:"High Resolution Relative Seconds.vi"() -> ("relative seconds"=w448:dbl)
                  }
                  frame #1 {
                    # "zyx"
                    # "スライス像を段々ずらしで重ねる"
                    n104 = for {
                      tunnel: w463 -> [w482] mode=indexing
                      tunnel: [w479] -> w460 mode=indexing
                      tunnel: w462 -> [w478]
                      tunnel: w461 -> [w477]
                      workers-P: _ -> [_]
                      i -> [w481]
                      n105 = Compound Arithmetic op=MULTIPLY(w481, w478) -> (w480:dbl)
                      n106 = case shown="False" w477 {
                        tunnel: w482 -> [w489 w507]
                        tunnel: w480 -> [w492 w506]
                        tunnel: [w483 w505] -> w479
                        frame False {
                          n107 = Array Size(array=w489) -> (size(s)=w488:i32[])
                          n108 = Index Array(array=w488) -> (element #2=w487:i32)  [unwired: 2 in, 1 out]
                          n109 = for {
                            N: w487 -> [_]
                            tunnel: [w493] -> w485 mode=indexing
                            i -> [w493]
                          }
                          n110 = Quotient & Remainder(x=w492, y=1.0) -> (x-y*floor(x/y)=w486:dbl, floor(x/y)=w490:dbl)
                          n111 = Subtract(x=w485, y=w486) -> (x-y=w484:dbl[])
                          n112 = for {